vi "initImageCluster.vi"() -> (1 "output cluster":T2)   [LabVIEW 2012]
uses:
  <vilib>/vision/Image Controls.llb/IMAQ Image.ctl
  GlobalBaslerCamera.vi
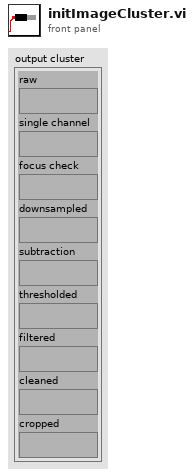
[diagram p1: front panel]
types:
  T1 = typedef "IMAQ Image.ctl" = refnum<image>
  T2 = cluster{"raw":T1, "single channel":T1, "focus check":T1, "downsampled":T1, "subtraction":T1, "thresholded":T1, "filtered":T1, "cleaned":T1, "cropped":T1}
  T3 = typedef "Image Type" = u32
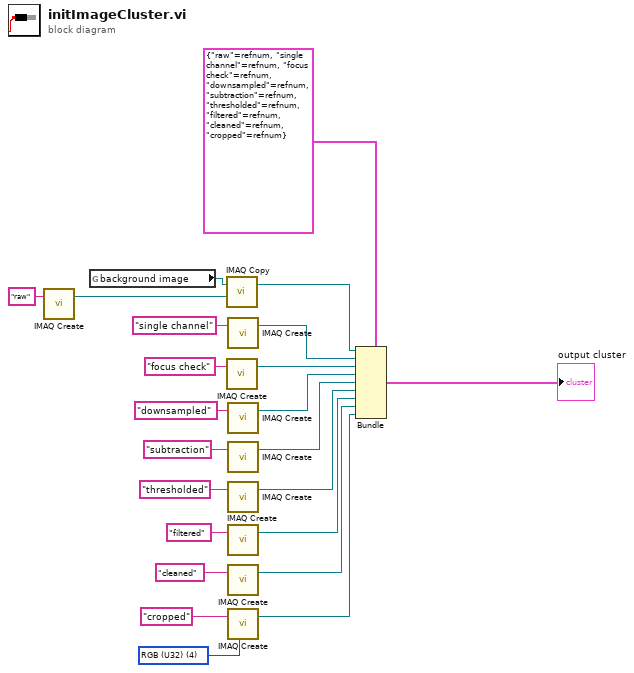
[diagram p0: block diagram]
diagram:
  w22 = T3 4 items=["Grayscale (U8)", "Grayscale (I16)", "Grayscale (SGL)", "Complex (CSG)", "RGB (U32)", "HSL (U32)", "RGB (U64)", "Grayscale (U16)"] ("Image Type")
  n1 = call "IMAQ Create"("Image Name"="raw") -> ("New Image"=w3:T1)  [unwired: 3 in, 2 out]
  n2 = global read "GlobalBaslerCamera.vi" "background image"() -> (w1:T1)
  n3 = call "IMAQ Copy"("Image Dst"=w3, "Image Src"=w1) -> ("Image Dst Out"=w2:T1)  [unwired: 4 in, 1 out]
  n4 = call "IMAQ Create"("Image Name"="focus check") -> ("New Image"=w11:T1)  [unwired: 3 in, 2 out]
  n5 = call "IMAQ Create"("Image Name"="single channel") -> ("New Image"=w12:T1)  [unwired: 3 in, 2 out]
  n6 = call "IMAQ Create"("Image Name"="downsampled") -> ("New Image"=w10:T1)  [unwired: 3 in, 2 out]
  n7 = call "IMAQ Create"("Image Name"="subtraction") -> ("New Image"=w5:T1)  [unwired: 3 in, 2 out]
  n8 = call "IMAQ Create"("Image Name"="thresholded") -> ("New Image"=w6:T1)  [unwired: 3 in, 2 out]
  n9 = call "IMAQ Create"("Image Name"="filtered") -> ("New Image"=w7:T1)  [unwired: 3 in, 2 out]
  n10 = call "IMAQ Create"("Image Name"="cleaned") -> ("New Image"=w8:T1)  [unwired: 3 in, 2 out]
  n11 = call "IMAQ Create"("Image Name"="cropped", "Image Type"=w22) -> ("New Image"=w9:T1)  [unwired: 2 in, 2 out]
  n12 = Bundle(cluster=T2 {"raw"="raw", "single channel"="single channel", "focus check"="focus check", "downsampled"="downsampled", "subtraction"="subtraction", "thresholded"="thresholded", "filtered"="filtered", "cleaned"="cleaned", "cropped"="cropped"} ("image cluster out"), "raw"=w2, "single channel"=w12, "focus check"=w11, "downsampled"=w10, "subtraction"=w5, "thresholded"=w6, "filtered"=w7, "cleaned"=w8, "cropped"=w9) -> (→"output cluster":T2)
